vi "HFRR ADV v044.vi"() -> ()   [LabVIEW 2025] (continued)
  # "Calibration failed. The measured stroke length differs from the factory calibration value by more than 20%. Please perform the calibration again."
  # "Step 1 — Ball Holder"
  # "Remove the ball holder by loosening and removing the center screw for Friction calibration."
  # "Step 2 — Disc Holder"
  # "Remove the disc holder by loosening and removing the opposing screws. Clean any fluid present in the disc holder."
  # "Step 3 — Calibration Head"
  # "Place the calibration holder in position and securely tighten the center screw."
  # "Step 4 — Calibration Holder"
  # "Place the calibration holder in position and tighten the two securing screws"
  # "Step 5 — Tare (Spring at Free Length)"
  # "Ensure the spring is at its contact (compressed) length — the micrometer head is in contact. Click Tare Sensor to zero the friction force baseline."
  # "Step 6 — Measure Friction Force"
  # "Run the Actual Test to measure Friction Force."
  # "Calibration in Progress"
  # "Step 7 — CALIBRATION RESULT"
  # "Calibration completed successfully. The measured friction force is within the acceptable tolerance range of the factory calibration value."
  # "Calibration failed. The measured friction force differs from the factory calibration value . Please perform the calibration again."
  # "Spring Constant: k = 1.000 N/mm\nSpring force |F| = k Ч d"
  # "Calibrates the sample/bath temperature sensor. \nUsed for test specimen and lubricant temperature measurement."
  # "Calibrates the ambient air temperature sensor. \nUsed for environmental chamber monitoring."
  # "Set B\n60 °C\nHigh-point calibration"
  # "Set A\n0 °C\nIce-point calibration"
  # "Set B\n60 °C\nHigh-point calibration"
  # "Set A\n0 °C\nIce-point calibration"
  # "Select Temperature Sensor"
  # "Choose which temperature sensor you are calibrating. Both use the same two-\npoint procedure: 0 °C (ice-point) and 60 °C (high-point)."
  # "Step 1 — Reference Instrument Setup"
  # "Connect a calibrated reference to the DUT port. This calibration performs two sets: one at 0 °C and one at 60 °C."
  # "Set A\n0 °C\nIce-point calibration"
  # "Set B\n60 °C\nHigh-point calibration"
  # "Allow the temperature bath to stabilise for at least 2 minutes at each set-point before recording the reading."
  # "Step 2 — Set A:  0 °C Calibration"
  # "Connect the  0 °C reference connector. Wait for the temperature to stabilise. Once stable, and click Record Point."
  # "Step 3 — Set B:  60 °C Calibration"
  # "Connect the  60 °C reference connector. Wait for the temperature to stabilise. Once stable, and click Record Point."
  # "Sample Temperature Calibration Complete"
  # "Sample Temperature Calibration PASSED\nMax deviation 0.200 °C — within ±0.5 °C tolerance. Two-point correction applied (0 °C & 60 °C)."
  # "Sample  Temperature Calibration Failed\nmeasured Sample Temperature differs from the factory calibration value"
  # "Step 1 — Reference Instrument Setup"
  # "Connect a calibrated reference to the DUT port. This calibration performs two sets: one at 0 °C and one at 60 °C."
  # "Set A\n0 °C\nIce-point calibration"
  # "Set B\n60 °C\nHigh-point calibration"
  # "Allow the temperature bath to stabilise for at least 2 minutes at each set-point before recording the reading."
  # "Step 2 — Set A:  0 °C Calibration"
  # "Connect the  0 °C reference connector. Wait for the temperature to stabilise. Once stable, and click Record Point."
  # "Step 3 — Set B:  60 °C Calibration"
  # "Connect the  60 °C reference connector. Wait for the temperature to stabilise. Once stable, and click Record Point."
  # "Air Temperature Calibration Complete"
  # "Air Temperature Calibration PASSED\nMax deviation 0.200 °C — within ±0.5 °C tolerance. Two-point correction applied (0 °C & 60 °C)."
  # "Air  Temperature Calibration Failed\nmeasured Sample Temperature differs from the factory calibration value"
  # "System Control Commands\nS;1 - Starts the full automation cycle (Runs Priming-humidify till 70RH sequence first, then switches to Maintenance).\nS;0 - Stops the system immediately and enters Standby mode (Safe State: All actuators OFF).\nM;1 - Skips the priming sequence and jumps directly to Maintenance mode (PID control).\nR;1 - Resets the logic state machine and clears all errors, returning to Standby.\nService Mode (Manual Control)\nX;1 - Enters Manual Service Mode. This disables all automatic logic, sensor safety checks, and timers.\nX;0 - Exits Manual Service Mode and returns to Standby (Safe State).\nActuator Commands (Only work after sending X;1)\nP;[0-255] - Sets the Pump PWM. Note that this is Active Low (0 = Max Flow, 255 = Pump OFF).\nF;I;[0-255] - Sets the Intake Fan speed (0 = OFF, 255 = Max Speed).\nF;O;[0-255] - Sets the Exhaust Fan speed (0 = OFF, 255 = Max Speed).\nD;1 - Turns the Dehumidifier Relay ON.\nD;0 - Turns the Dehumidifier Relay OFF."
  # "%RH"
types:
  T1 = enum32{"Home", "Dashboard", "Imaging", "Report", "Analysis", "About", "Test Setup", "Advance", "Calibration"}
  T2 = typedef "imagedata.ctl" = cluster{"image type":i32, "image depth":i32, "image":u8[], "mask":u8[], "colors":u32[], "Rectangle":cluster{"left":i16, "top":i16, "right":i16, "bottom":i16}}
  T3 = enum32{"HOME", "Test Setup", "Acquire", "Compare Files", "Print Report", "About", "Advance", "Mooha"}
  T4 = enum32{"HOME", "Test Setup", "Acquire", "Adv Scar", "Adv Scar Report", "Compare Files", "Calibration", "About", "Advance", "Mooha"}
  T5 = enum16{"ASTM D6079", "ISO 12156", "CEC F-096-A-06", "Custom"}
  T6 = enum32{"Dashboard 1", "Dashboard 2", "Dashboard 3"}
  T7 = enum32{"COF", "Friction", "ECR", "Temperature", "Stroke"}
  T8 = enum32{"Coefficient Of Friction", "Air Temperature", "Humidity", "Stroke", "Sample Temperature", "Electrical Contact Resistance", "Frequency", "Air Temp vs Rh"}
  T9 = enum32{"Main", "Stroke", "Friction", "Temperature"}
  T10 = enum32{"Stroke Calibration", "Friction Force Calibration", "Temperature Calibration", "Default"}
  T11 = enum32{"Step 1", "Step 2", "Step 3", "Step 4", "Step 5", "Step 6", "Step 7", "Step 8", "Step 9"}
  T12 = enum32{"Test Progress", "Stroke Points Completed"}
  T13 = enum32{"Page 1", "Page 2", "Page 3", "Page 4", "Page 5", "Page 6"}
  T14 = enum32{"Main", "Step 1", "Step 2", "Step 3", "Step 4", "Air Step 1", "Air Step 2", "Air Step 3", "Air Step 4"}
  T15 = enum32{"Air Temperature", "Sample Temperature", "Default"}
  T16 = enum32{"COMMUNICATION", "CALIBRATION", "Temp Variables", "Camera", "WO 2472 (1)", "WO 2472 (2)", "WO 2472 (3)"}
  T17 = typedef "Auto Start enum.ctl" = enum16{"Init", "Humidity & Temperature On", "Reach point", "Maintain Stage", "Start Stage", "close", "Exit"}
  T18 = cluster{"Read Heave and Surge":string, "Bytes at Heave Port":dbl, "Heave and Surge COM Port:":refnum<visa-resource-name>, "Com Port 2":refnum<visa-resource-name>, "Residual Due":string, "Heave COM Status 2":bool, "Heave COM Status":bool, "Port 2":bool, "Sway PPR":dbl, "Surge PPR":dbl, "Heave PPR":dbl, "Sway Pitch":dbl, "Surge Pitch":dbl, "Heave Pitch":dbl, "Sway Pulses/mm":dbl, "Surge Pulses/mm":dbl, "Heave Pulses/mm":dbl, "inner loop":dbl, "Read Heave and Surge 2":string, "String 36":string, "Write S":bool, "WriteCC1":string[], "Heave COM Loop":i32, "LastCom":string, "EXIT":bool, "Error Heave":errorcluster}
  T19 = enum8{"Enabled", "Disabled", "Disabled and Grayed Out"}
  T20 = cluster{"Read Uno":string, "Bytes at Heave Port":dbl, "UNO COM Port:":refnum<visa-resource-name>, "UNO COM Port: 2":refnum<visa-resource-name>, "Residual Due":string, "UNO COM Status 2":bool, "UNO COM Status":bool, "Port 2":bool, "Sway PPR":dbl, "Surge PPR":dbl, "Heave PPR":dbl, "Sway Pitch":dbl, "Surge Pitch":dbl, "Heave Pitch":dbl, "Sway Pulses/mm":dbl, "Surge Pulses/mm":dbl, "Heave Pulses/mm":dbl, "inner loop":dbl, "Read Heave and Surge 2":string, "String 36":string, "Write S":bool, "WriteCC1":string[], "Heave COM Loop":i32, "LastCom":string, "EXIT":bool, "Error Heave":errorcluster}
  T21 = enum32{"HOME", "Test Setup", "Acquire", "Adv Scar", "Adv Scar Report", "Compare Files", "About", "Advance", "Mooha"}
  T22 = typedef "POST ANALYSIS ENUM.ctl" = enum16{"OPEN EXE", "INIT", "OPEN FILE", "FIT", "DRAW REC", "DRAW LINE", "PAN", "ZOOM IN", "ZOOM OUT", "SET ZOOM", "CLEAR ROI", "GET MEASUREMENTS", "RESIZE MODE", "STREAM START", "STREAM STOP", "SHOW UI", "MINIMIZE UI", "HIDE UI", "CKISE APP", "CLOSE CONNECTION", "SAVE IMAGE", "SET ROI COLOR", "READ", "TCP CHECK", "CLOSE"}
  T23 = typedef "CAMERA LIVE FEED ENUM.ctl" = enum16{"OPEN EXE", "INIT", "READ", "CAMERA CONNECT", "CAMERA START", "CAMERA STOP", "CAMERA GRAY", "CAMERA RGB", "CAMERA MINIMIZE", "CAMERA CLOSE", "CAMERA MODE LIST", "CAMERA MODE SET", "CAMERA RESTORE", "CAMERA SAVE", "CLOSE"}
  T24 = enum16{"Always On", "Always Off", "Off While Running"}
  T25 = enum32{"Home", "Dashboard", "Imaging", "Report", "Analysis", "About", "Test Setup", "Advance"}
  T26 = cluster{"File Name":string, "Test Method":string, "Operator":string, "Fuel Description":string, "Date and time":string}
  T27 = enum32{"Home", "Dashboard", "Imaging", "Report", "Analysis", "About", "Test Setup"}
  T28 = enum32{"HOME", "Test Setup", "Acquire", "Compare Files", "About", "Advance", "Mooha"}
  T29 = typedef "NI_ReportGenerationCore.lvlib/HTML Report Image Alignment.ctl" = enum16{"(default)", "LEFT", "RIGHT", "TOP", "TEXTTOP", "MIDDLE", "ABSMIDDLE", "BASELINE", "BOTTOM", "ABSBOTTOM"}
  T30 = cluster{"y":dbl, "LVDT STROKE DISPLAY":dbl, "y":dbl}
  T31 = enum16{"INIT", "READ", "MANUAL WRITE", "WRITE", "CLOSE", "ERROR INIT"}
diagram:
  w1 = FALSE
  w8 = 0.0 ("ch0_filt")
  w10 = -9999999.0 ("max_ch0")
  w11 = 9999999.0 ("min_ch0")
  w22 = FALSE ("Visible")
  w23 = T19."Enabled" ("Disabled")
  w26 = FALSE ("Visible")
  w25 = FALSE ("Humidity Off Command")
  w41 = "" ("USER ID")
  (unwired) T21."HOME" ("Main Tab")
  # "Temperature Continue Air Step 2"
  # "[CH1]    - FF\n[CH2]   - TEMPERATURE\n[CH3]    - Humidity\n[CH4]    - AIR TEMP\n[CH5]\\- Visa Uno\n[CH6] \\- Visa Due\n[CH7]  \\- file path\n[CH8]   - Displacement Gain\n[CHA]   - Stroke Gain\n[CHB]   - Stroke PID Gain\n[CHC]   -Language Selection\n[CHD]   -Power +\n[CHE]   -Power_\n[CHF]   -Heater\n[CHG]   -Humidity Wet\n[CHH]   -Humidity Dry\n[CHI]   -Integral Time \n[CHIJ   -Air intercept\n[CHI]   -Temp Intercept"
  n1 = local write "Cal Password"("" ("Cal Password")) -> ()
  n2 = property on="Auto Start Test" class="Bool (strict)"("Visible"=TRUE) -> ()  [unwired: 2 in, 2 out]
  n3 = property on="Friction Force Calibration Result Tab" class="TabCtl (strict)"("Visible"=FALSE) -> ()  [unwired: 2 in, 2 out]
  n4 = property on="FRICVALZ 2" class="Bool (strict)"("DisabledEnum"=w23) -> ()  [unwired: 2 in, 2 out]
  n5 = property on="FRICVALZ 4" class="Bool (strict)"("DisabledEnum"=w23) -> ()  [unwired: 2 in, 2 out]
  n6 = property on="FRICVALZ 3" class="Bool (strict)"("DisabledEnum"=w23) -> ()  [unwired: 2 in, 2 out]
  n7 = property on="About" class="Clust (strict)"("Visible"=FALSE) -> ()  [unwired: 2 in, 2 out]
  n8 = property on="Wrong Password" class="Str"("Visible"=w22) -> ()  [unwired: 2 in, 2 out]
  n9 = property on="Calibration 2" class="TabCtl (strict)"("Visible"=w22) -> ()  [unwired: 2 in, 2 out]
  n10 = local write "Temperature Selection"(T15."Default" ("Temperature Selection")) -> ()
  n11 = flat-sequence {
    tunnel: [w70] -> w7
    tunnel: [w115] -> w33
    tunnel: w7 -> [w110]
    tunnel: [w116] -> w35
    tunnel: w33 -> [w116]
    tunnel: w35 -> [w176]
    tunnel: [w176] -> w34
    tunnel: w34 -> [w207]
    tunnel: [w207] -> w44
    tunnel: w44 -> [w214]
    tunnel: [w220] -> w32
    tunnel: [w208] -> w31
    tunnel: [w262] -> w6
    tunnel: [w261] -> _
    tunnel: w32 -> [w261]
    tunnel: w31 -> [w262]
    frame #0 {
      n12 = call "CLOSE CONNECTION.vi"("error in (no error)"="error in (no error) 2") -> ("error out"=w75:errorcluster)  [unwired: 10 in]
      n13 = call <vilib>:"Clear Errors.vi"("error in (no error)"=w75) -> ("error out"=w74:errorcluster)  [unwired: 5 in, 1 out]
      n14 = disable-structure shown="Enabled" {
        disable-tunnel: w74 -> [w102 _]
        disable-tunnel: [w101 _] -> w73
        frame Enabled {
          n15 = call <userlib>:"Fit VI window to Largest Dec.vi"("error in (no error)"=w102, "border spacing (2 px)"=1) -> ("error out"=w105:errorcluster, "dup VI Ref"=w109:refnum<vi>)  [unwired: 4 in]
          n16 = invoke on="Invoke Node" class="VI" method="FP.Run-Time Position.Maximized"(reference=w109, error in=w105) -> (error out=w106:errorcluster)  [unwired: 2 in, 3 out]
          n17 = call <vilib>:"Clear Errors.vi"("error in (no error)"=w106) -> ("error out"=w108:errorcluster)  [unwired: 5 in, 1 out]
          n18 = control-ref of="This VI"() -> (w100:refnum<vi>)
          n19 = invoke on="Invoke Node" class="VI" method="Default Vals.Reinit All"(reference=w100, error in=w108) -> (reference out=w104:refnum<vi>, error out=w103:errorcluster)  [unwired: 1 in, 1 out]
          n20 = Close Reference(reference=w104, error in (no error)=w103) -> (error out=w101:errorcluster)
        }
        frame Disabled {
        }
      }
      n21 = call "Stall Data Flow.vim"("value in"=w73, "milliseconds to wait"=u32 2000) -> ("value out"=w72:errorcluster)  [unwired: 1 out]
      n22 = call "Read Config.vi"("error in (no error)"=w72) -> ("error out"=w70:errorcluster, "STROKE PARAMETERS"=w81:dbl[], "ADC PARAMETERS"=w82:dbl[], "PID  PARAMETERS"=w83:dbl[], "CALIBRATION PARAMETERS"=w68:string[], "Stroke Calibration"=w80:string)  [unwired: 5 in]
      n23 = Index Array(array=w81) -> (element #1=w98:dbl, element #2=w99:dbl)  [unwired: 2 in]
      n24 = Index Array(array=w68) -> (element #1=w67:string, element #2=w66:string, element #3=w65:string, element #4=w64:string, element #5=w63:string)  [unwired: 5 in]
      n25 = Index Array(array=w82) -> (element #1=w94:dbl, element #2=w95:dbl, element #3=w96:dbl, element #4=w97:dbl, element #5=w62:dbl)  [unwired: 5 in]
      n26 = Index Array(array=w83) -> (element #1=w85:dbl, element #2=w86:dbl, element #3=w87:dbl, element #4=w88:dbl, element #5=w89:dbl, element #6=w90:dbl, element #7=w91:dbl, element #8=w92:dbl, element #9=w93:dbl)  [unwired: 9 in]
      n27 = local write "STROKE FILTER"(w98) -> ()
      n28 = local write "Add up Stroke"(w99) -> ()
      n29 = local write "milliseconds to wait"(w85) -> ()
      n30 = local write "dt"(w86) -> ()
      n31 = local write "kp"(w87) -> ()
      n32 = local write "ki"(w88) -> ()
      n33 = local write "kd"(w89) -> ()
      n34 = local write "max_step_change"(w90) -> ()
      n35 = local write "max_amplitude"(w91) -> ()
      n36 = local write "min_amplitude"(w92) -> ()
      n37 = local write "startup_cmd"(w93) -> ()
      n38 = local write "VREF"(w94) -> ()
      n39 = local write "ADC_Resolution"(w95) -> ()
      n40 = local write "PIEZO_CAL_FACTOR"(w96) -> ()
      n41 = local write "NORMAL_FORCE"(w97) -> ()
      n42 = local write "Machine Serial Number"(w63) -> ()
      n43 = local write "STROKE CALIBRATION"(w67) -> ()
      n44 = local write "FRICTION CALIBRATION"(w66) -> ()
      n45 = local write "TEMPERATURE CALIBRATION"(w65) -> ()
      n46 = Fract/Exp String To Number(string=w64) -> (number=w69:dbl)  [unwired: 3 in, 1 out]
      n47 = local write "FF CAL EXCPTED VALUE"(w62) -> ()
      n48 = Spreadsheet String To Array(delimiter (Tab)=";", format string="", spreadsheet string=w80, array type (2D Dbl)=dbl[] []) -> (array=w84:dbl[])
      n49 = local write "Temperature diff"(w69) -> ()
      n50 = local write "calibration values"(w84) -> ()
    }
    frame #1 {
      n51 = property on="Auto Scar Check" class="Clust (strict)"("Visible"=TRUE) -> ()  [unwired: 2 in, 2 out]
      n52 = property on="Sign In" class="Bool (strict)"("DisabledEnum"=T19."Disabled" ("Disabled")) -> ()  [unwired: 2 in, 2 out]
      n53 = local write "sign in temp"(FALSE ("sign in temp")) -> ()
      n54 = call "dialog box.vi"("Status"="Before starting the test, verify that the microscope cable is connected.", "error in"=w110) -> ("error out"=w115:errorcluster)  [unwired: 8 in]
    }
    frame #2 {
      (unwired) TRUE ("Re-Initialise")
      # "kkkkk"
      # "C:\\Windows\\wndcm_pw_stdED hfrr.txt"
      # "C:\\LAB-IQ NXT"
      # "C:\\LAB-IQ NXT\\wndcm_pw_stdED hfrr.txt"
      # "password file"
      n55 = Current VI's Path() -> (path=w132:path)
      n56 = Strip Path(path=w132) -> (stripped path=w125:path)  [unwired: 1 out]
      n57 = local write "main tab sub"(enum32{"Page 1", "Page 2"}."Page 1" ("main tab sub")) -> ()
      n58 = local write "Main Tab Display"(T6."Dashboard 1" ("Main Tab Display")) -> ()
      n59 = local write "Main Tab"(T4."HOME" ("Main Tab")) -> ()
      n60 = Path To String(path=w125) -> (string=w127:string)
      n61 = Search/Split String(string=w127, search string/char (-)=".exe") -> (match + rest of string=w129:string)  [unwired: 1 in, 2 out]
      n62 = Match True/False String(2:".vi" ("false string"), 3:".exe" ("true string"), 4:w129) -> (0:w126:bool)  [unwired: 1 out]
      n63 = List Folder(path=path "C:/LAB-IQ" ("directory path"), pattern="*.txt") -> (filenames=w138:string[])  [unwired: 2 in, 3 out]
      n64 = case shown="True" w126 {
        tunnel: w125 -> [w147 w149]
        tunnel: [w147 w148] -> w123
        frame False {
        }
        frame True {
          n65 = Strip Path(path=w149) -> (stripped path=w148:path)  [unwired: 1 out]
        }
      }
      n66 = Search 1D Array(1D array=w138, element="wndcm_pw_stdED hfrr.txt") -> (index of element=w141:i32)  [unwired: 1 in]
      n67 = Equal?(x=w141, y=-1) -> (x = y?=w136:bool)
      n68 = Path To String(path=w123) -> (string=→"Gain path":string)
      n69 = case shown="True" w136 {
        frame False {
        }
        frame True {
          n70 = String To Byte Array(string="123\n") -> (unsigned byte array=w154:u8[])
          n71 = Array Size(array=w154) -> (size(s)=w153:i32)
          n72 = for {
            N: w153 -> [_]
            tunnel: w154 -> [w167]
            tunnel: [w164] -> w156 mode=indexing
            tunnel: w153 -> [w159]
            i -> [w157]
            n73 = Decrement(x=w159) -> (x-1=w160:i32)
            n74 = Index Array(array=w167, index=w157) -> (element=w166:u8)
            n75 = Equal?(x=w157, y=w160) -> (x = y?=w161:bool)
            n76 = Number To Decimal String(number=w166) -> (decimal integer string=w165:string)  [unwired: 1 in]
            n77 = Select(t="", s=w161, f="\r") -> (s? t:f=w158:string)
            n78 = Concatenate Strings(w165, w158) -> (w164:string)
          }
          n79 = local read "file path"() -> (w150:path)
          n80 = Concatenate Strings(w156) -> (w152:string)
          n81 = call <vilib>:"Write Characters To File.vi"("append to file? (new file:F)"=FALSE, "character string"=w152, "file path (dialog if empty)"=w150) -> ()  [unwired: 2 in, 1 out]
        }
      }
      n82 = local write "conststatus"(0.0 ("rpm value : 2")) -> ()
      n83 = local write "EVENT LOG"("") -> ()
      n84 = local write "COUNT"(0 ("COUNT")) -> ()
      n85 = local write "clk"(0.0 ("clk")) -> ()
      n86 = local write "Flag"(0.0 ("Flag")) -> ()
      n87 = local write "Lan flag"(0.0 ("Lan flag")) -> ()
      n88 = local write "Com flag"(u32 0 ("Com flag")) -> ()
      n89 = local write "refresh flag"(FALSE ("refresh flag")) -> ()
      "file path" <- path "C:/LAB-IQ/wndcm_pw_stdED hfrr.txt" ("file path")
      "FF buffer" <- dbl[] [] ("FF buffer")
    }
    frame #3 {
      # "C:\\WinDucom\\calibrate WO 2391.dcf"
      n90 = String To Path(string="C:\\LAB-IQ\\Image Calibrate v01.dcf") -> (path=w171:path)
      n91 = String To Path(string="C:\\LAB-IQ\\calibrate WO 2472.dcf") -> (path=w175:path)
      n92 = Open/Create/Replace File "Open File"(file path (use dialog)=w175) -> (refnum out=w174:refnum<file>)  [unwired: 5 in, 2 out]
      n93 = Open/Create/Replace File ("Open File")(file path (use dialog)=w171) -> (refnum out=w170:refnum<file>)  [unwired: 5 in, 2 out]
      n94 = for {
        N: 4 -> [_]
        tunnel: w170 -> [w182]
        i -> [w178]
        n95 = Read from Text File ("Read File")(file (use dialog)=w182) -> (text=w183:string)  [unwired: 3 in, 3 out]
        n96 = String Subset(string=w183, offset (0)=6, length (rest)=10 ("length (rest)")) -> (substring=w179:string)
        n97 = Fract/Exp String To Number(string=w179) -> (number=w177:dbl)  [unwired: 3 in, 1 out]
        n98 = case shown="3" w178 {
          tunnel: w177 -> [w184 w185 _ w186 _]
          frame 0 {
            n99 = local write "5x Gain"(w184) -> ()
          }
          frame 1 {
            n100 = local write "10x Gain"(w185) -> ()
          }
          frame 2 {
          }
          frame 3 {
            n101 = local write "100x gain"(w186) -> ()
          }
          frame 4, Default {
          }
        }
      }
      n102 = for {
        N: 24 -> [_]
        tunnel: w174 -> [w195]
        i -> [w189]
        (unwired) TRUE ("line mode (F)")
        n103 = Read from Text File "Read File"(file (use dialog)=w195) -> (text=w194:string)  [unwired: 3 in, 3 out]
        n104 = Match Pattern(string=w194, regular expression="]") -> (after substring=w192:string)  [unwired: 1 in, 3 out]
        n105 = String Subset(string=w194, offset (0)=5, length (rest)=10 ("length (rest)")) -> (substring=w187:string)
        n106 = Fract/Exp String To Number(string=w187) -> (number=w188:dbl)  [unwired: 3 in, 1 out]
        n107 = Match Pattern(string=w192, regular expression="-") -> (before substring=w190:string)  [unwired: 1 in, 3 out]
        n108 = case shown="18" w189 {
          tunnel: w188 -> [_ _ _ _ _ _ _ _ _ _ w202 _ _ _ _ _ _ _ _ _ _ _ _ _ _]
          tunnel: w190 -> [_ _ _ _ w198 w199 w200 _ _ _ _ _ _ _ _ _ _ _ _ _ w203 _ w204 w205 _]
          frame 0 {
          }
          frame 1 {
          }
          frame 2 {
          }
          frame 3 {
          }
          frame 4 {
            n109 = local write "Com Port 1"(w198) -> ()
          }
          frame 5 {
            n110 = local write "Com Port 2"(w199) -> ()
            n111 = local write "visa due"(w199) -> ()
          }
          frame 6 {
            n112 = String To Path(string=w200) -> (path=w201:path)
            n113 = local write "File Path"(w201) -> ()
          }
          frame 7 {
          }
          frame 8 {
          }
          frame 9 {
          }
          frame 10 {
            n114 = local write "Language Selection"(w202) -> ()
          }
          frame 11 {
          }
          frame 12 {
          }
          frame 13 {
          }
          frame 14 {
          }
          frame 15 {
          }
          frame 16 {
          }
          frame 17 {
          }
          frame 18 {
          }
          frame 21 {
          }
          frame 22 {
            n115 = local write "Com Port 3"(w203) -> ()
          }
          frame 23 {
          }
          frame 19 {
            n116 = local write "C3 :"(w204) -> ()
          }
          frame 20 {
            n117 = local write "Camera Port :"(w205) -> ()
          }
          frame 24, Default {
          }
        }
      }
    }
    frame #4 {
      n118 = Wait (ms)(milliseconds to wait=u32 1000) -> ()  [unwired: 1 out]
    }
    frame #5 {
      w223 = u32 2000 ("milliseconds to wait")
      w250 = u32 2000 ("milliseconds to wait")
      n119 = call "CAMERA LIVE FEED FGV.vi"("Enum - Menu"=CAMERA_LIVE_FEED_ENUM."OPEN EXE", "error in (no error)"=w214) -> ("error out"=w256:errorcluster)  [unwired: 8 in, 1 out]
      n120 = call "IMAGE ANALYSIS.vi"("Enum"=POST_ANALYSIS_ENUM."OPEN EXE", "error in"=w214) -> ("error out"=w211:errorcluster)  [unwired: 8 in, 1 out]
      n121 = call "Stall Data Flow.vim"("value in"=w256, "milliseconds to wait"=w250) -> ("value out"=w254:errorcluster)  [unwired: 1 out]
      n122 = call "Stall Data Flow.vim"("value in"=w211, "milliseconds to wait"=u32 8000) -> ("value out"=w210:errorcluster)  [unwired: 1 out]
      n123 = call "CAMERA LIVE FEED FGV.vi"("Enum - Menu"=CAMERA_LIVE_FEED_ENUM."INIT", "error in (no error)"=w254) -> ("error out"=w252:errorcluster)  [unwired: 8 in, 1 out]
      n124 = call "IMAGE ANALYSIS.vi"("Enum"=POST_ANALYSIS_ENUM."INIT", "error in"=w210) -> ("error out"=w208:errorcluster)  [unwired: 8 in, 1 out]
      n125 = case shown="Error .." w252 {
        selector: w252 -> [w257 _]
        tunnel: [w257 _] -> w251
        frame No Error {
        }
        frame Error {
          n126 = One Button Dialog(message="Camera initialization error.\nPlease Restart the software") -> ()  [unwired: 1 in, 1 out]
        }
      }
      n127 = property on="Camera Port :" class="CmbBox"() -> ("Strings[]"=w248:string[], "Value"=w249:string)  [unwired: 2 in, 2 out]
      n128 = Search 1D Array(1D array=w248, element=w249) -> (index of element=w247:i32)  [unwired: 1 in]
      n129 = Type Cast(type=30, x=w247) -> (*(type *) &x=w245:i32)
      n130 = call "Stall Data Flow.vim"("value in"=w251, "milliseconds to wait"=w250) -> ("value out"=w227:errorcluster)  [unwired: 1 out]
      n131 = Add(x=w245, y=48) -> (x+y=w226:i32)
      n132 = call "CAMERA LIVE FEED FGV.vi"("Enum - Menu"=CAMERA_LIVE_FEED_ENUM."CAMERA CONNECT", "error in (no error)"=w227, "CAMERA PORT"=w226) -> ("error out"=w236:errorcluster)  [unwired: 7 in, 1 out]
      n133 = call "Stall Data Flow.vim"("value in"=w236, "milliseconds to wait"=u32 5000) -> ("value out"=w237:errorcluster)  [unwired: 1 out]
      n134 = call "CAMERA LIVE FEED FGV.vi"("Enum - Menu"=CAMERA_LIVE_FEED_ENUM."CAMERA MODE LIST", "error in (no error)"=w237) -> ("error out"=w239:errorcluster)  [unwired: 8 in, 1 out]
      n135 = call "Stall Data Flow.vim"("value in"=w239, "milliseconds to wait"=w223) -> ("value out"=w238:errorcluster)  [unwired: 1 out]
      n136 = call "CAMERA LIVE FEED FGV.vi"("Enum - Menu"=CAMERA_LIVE_FEED_ENUM."READ", "error in (no error)"=w238) -> ("error out"=w225:errorcluster, "data out"=→"Camera List":string)  [unwired: 8 in]
      n137 = Type Cast(type=30, x=0) -> (*(type *) &x=w219:i32)
      n138 = call "Stall Data Flow.vim"("value in"=w225, "milliseconds to wait"=w223) -> ("value out"=w224:errorcluster)  [unwired: 1 out]
      n139 = Add(x=w219, y=48) -> (x+y=w217:i32)
      n140 = call "CAMERA LIVE FEED FGV.vi"("Enum - Menu"=CAMERA_LIVE_FEED_ENUM."CAMERA MODE SET", "error in (no error)"=w224, "CAMERA MODE"=w217) -> ("error out"=w221:errorcluster)  [unwired: 7 in, 1 out]
      n141 = call "Stall Data Flow.vim"("value in"=w221, "milliseconds to wait"=u32 2000) -> ("value out"=w241:errorcluster)  [unwired: 1 out]
      n142 = call "CAMERA LIVE FEED FGV.vi"("Enum - Menu"=CAMERA_LIVE_FEED_ENUM."CAMERA START", "error in (no error)"=w241) -> ("error out"=w242:errorcluster)  [unwired: 8 in, 1 out]
      n143 = call "Stall Data Flow.vim"("value in"=w242, "milliseconds to wait"=u32 1000) -> ("value out"=w243:errorcluster)  [unwired: 1 out]
      n144 = call "CAMERA LIVE FEED FGV.vi"("Enum - Menu"=CAMERA_LIVE_FEED_ENUM."CAMERA MINIMIZE", "error in (no error)"=w243) -> ("error out"=w220:errorcluster)  [unwired: 8 in, 1 out]
    }
    frame #6 {
      n145 = case shown="No Error" w261 {
        frame No Error {
          n146 = property on="Auto Scar Check" class="Clust (strict)"("Visible"=FALSE) -> ()  [unwired: 2 in, 2 out]
        }
        frame Error {
        }
      }
      n147 = property on="Sign In" class="Bool (strict)"("DisabledEnum"=T19."Enabled" ("Disabled")) -> ()  [unwired: 2 in, 2 out]
      n148 = local write "sign in temp"(TRUE ("sign in temp")) -> ()
    }
  }
  n149 = local write "Calibration Selection"(T10."Default" ("Calibration Selection")) -> ()
  n150 = local write "SCAR MEASURMENT"(enum32{"Auto Scar", "Manual Scar"}."Manual Scar" ("SCAR MEASURMENT")) -> ()
  n151 = property on="Service Left" class="Bool (strict)"("Visible"=w1) -> ()  [unwired: 2 in, 2 out]
  n152 = property on="Service Right" class="Bool (strict)"("Visible"=w1) -> ()  [unwired: 2 in, 2 out]
  n153 = property on="Service Bottom" class="Bool (strict)"("Visible"=w1) -> ()  [unwired: 2 in, 2 out]
  n154 = local write "Temperature Off Command"(w25) -> ()
  n155 = local write "Main Dashboard Buttons"(T1."Home" ("Main Dashboard Buttons")) -> ()
  n156 = property on="Tab Control 6" class="TabCtl (strict)"("Visible"=FALSE) -> ()  [unwired: 2 in, 2 out]
  n157 = local write "Humidity Off Command"(w25) -> ()
  n158 = local write "CAMERA ROI MIN TEMP"(w25) -> ()
  n159 = local write "TEST FILE NAM,E SAVED"(w25) -> ()
  n160 = local write "LIVE FEED MIN TEMP"(w25) -> ()
  n161 = local write "SCAR MEASURMENT"(enum32{"Auto Scar", "Manual Scar"}."Manual Scar" ("SCAR MEASURMENT")) -> ()
  n162 = local write "Auto stop temp"(w26) -> ()
  n163 = local write "main tab sub"(enum32{"Page 1", "Page 2"}."Page 1" ("main tab sub")) -> ()
  n164 = while {
    stop <- w276 stop-if-true
    n165 = local read "Ambient Temperature"() -> (w274:dbl)
    n166 = local read "Sample Temperature 2"() -> (w273:dbl)
    n167 = Wait (ms)(milliseconds to wait=u32 200) -> ()  [unwired: 1 out]
    n168 = local write "Sensor value"(w274) -> ()
    n169 = local write "Sensor value"(w274) -> ()
    n170 = local write "Sensor value"(w273) -> ()
    n171 = local write "Sensor value"(w273) -> ()
    n172 = local write "Temperature — Live (Set A: 0 °C)"(w274) -> ()
    n173 = local write "Temperature — Live (Set A: 60 °C)"(w274) -> ()
    n174 = local write "Temperature — Live (Set A: 60 °C)"(w273) -> ()
    n175 = local write "Temperature — Live (Set A: 0 °C)"(w273) -> ()
    n176 = case shown="True" "Save Button" {
      selector: "Save Button" -> [_ w332]
      frame False {
      }
      frame True {
        n177 = Not(x=w332) -> (.not. x?=w331:bool)
        n178 = local read "Temperature diff"() -> (w328:dbl)
        n179 = local read "Machine Serial Number"() -> (w317:string)
        n180 = local read "milliseconds to wait"() -> (w364:u32)
        n181 = local write "Save Button"(w331) -> ()
        n182 = local read "max_step_change"() -> (w369:dbl)
        n183 = local read "FF CAL EXCPTED VALUE"() -> (w315:dbl)
        n184 = local read "max_amplitude"() -> (w370:dbl)
        n185 = local read "min_amplitude"() -> (w371:dbl)
        n186 = local read "PIEZO_CAL_FACTOR"() -> (w375:dbl)
        n187 = local read "startup_cmd"() -> (w372:dbl)
        n188 = local read "NORMAL_FORCE"() -> (w376:dbl)
        n189 = local read "ADC_Resolution"() -> (w374:dbl)
        n190 = local read "kp"() -> (w366:dbl)
        n191 = local read "kd"() -> (w368:dbl)
        n192 = local read "calibration values"() -> (w379:dbl[])
        n193 = local read "dt"() -> (w365:dbl)
        n194 = local read "ki"() -> (w367:dbl)
        n195 = local read "STROKE FILTER"() -> (w377:i32)
        n196 = local read "Add up Stroke"() -> (w378:dbl)
        n197 = Number To Fractional String(number=w328) -> (F-format string=w327:string)  [unwired: 3 in]
        n198 = local read "VREF"() -> (w373:dbl)
        n199 = Insert Into Array(array=dbl[] [], new element #1=w364, new element #2=w365, new element #3=w366, new element #4=w367, new element #5=w368, new element #6=w369, new element #7=w370, new element #8=w371, new element #9=w372) -> (w380:dbl[])  [unwired: 1 in]
        n200 = Insert Into Array(array=dbl[] [], new element #1=w373, new element #2=w374, new element #3=w375, new element #4=w376, new element #5=w315) -> (w381:dbl[])  [unwired: 1 in]
        n201 = Array To Spreadsheet String(delimiter (Tab)=";", array=w379, 3:"" ("format string")) -> (spreadsheet string=w383:string)
        n202 = Insert Into Array(array=dbl[] [], new element #1=w377, new element #2=w378) -> (w382:dbl[])  [unwired: 1 in]
        n203 = Insert Into Array(array=string[] [], new element #1="STROKE CALIBRATION", new element #2="FRICTION CALIBRATION", new element #3="TEMPERATURE CALIBRATION", new element #4=w327, new element #5=w317) -> (w329:string[])  [unwired: 1 in]
        n204 = call "Write Config.vi"("Stroke Calibration"=w383, "CALIBRATION PARAMETERS"=w329, "STROKE PARAMETERS"=w382, "ADC PARAMETERS"=w381, "PID  PARAMETERS"=w380) -> ("error out"=w362:errorcluster)  [unwired: 5 in, 1 out]
        n205 = call "Stall Data Flow.vim"("value in"=w362, "milliseconds to wait"=u32 2000) -> ("value out"=w363:errorcluster)  [unwired: 1 out]
        n206 = call "Read Config.vi"("error in (no error)"=w363) -> ("STROKE PARAMETERS"=w360:dbl[], "ADC PARAMETERS"=w359:dbl[], "PID  PARAMETERS"=w358:dbl[], "CALIBRATION PARAMETERS"=w323:string[], "Stroke Calibration"=w361:string)  [unwired: 5 in, 1 out]
        n207 = Index Array(array=w358) -> (element #1=w356:dbl, element #2=w355:dbl, element #3=w354:dbl, element #4=w353:dbl, element #5=w352:dbl, element #6=w351:dbl, element #7=w350:dbl, element #8=w349:dbl, element #9=w348:dbl)  [unwired: 9 in]
        n208 = Index Array(array=w359) -> (element #1=w347:dbl, element #2=w346:dbl, element #3=w345:dbl, element #4=w344:dbl, element #5=w314:dbl)  [unwired: 5 in]
        n209 = Index Array(array=w360) -> (element #1=w343:dbl, element #2=w342:dbl)  [unwired: 3 in, 1 out]
        n210 = Index Array(array=w323) -> (element #1=w320:string, element #2=w319:string, element #3=w318:string, element #4=w322:string, element #5=w316:string)  [unwired: 5 in]
        n211 = Spreadsheet String To Array(delimiter (Tab)=";", format string="", spreadsheet string=w361, array type (2D Dbl)=dbl[] []) -> (array=w357:dbl[])
        n212 = local write "STROKE CALIBRATION"(w320) -> ()
        n213 = local write "FRICTION CALIBRATION"(w319) -> ()
        n214 = local write "TEMPERATURE CALIBRATION"(w318) -> ()
        n215 = Fract/Exp String To Number(string=w322) -> (number=w321:dbl)  [unwired: 3 in, 1 out]
        n216 = local write "Machine Serial Number"(w316) -> ()
        n217 = local write "STROKE FILTER"(w343) -> ()
        n218 = local write "Add up Stroke"(w342) -> ()
        n219 = local write "VREF"(w347) -> ()
        n220 = local write "ADC_Resolution"(w346) -> ()
        n221 = local write "PIEZO_CAL_FACTOR"(w345) -> ()
        n222 = local write "NORMAL_FORCE"(w344) -> ()
        n223 = local write "FF CAL EXCPTED VALUE"(w314) -> ()
        n224 = local write "calibration values"(w357) -> ()
        n225 = local write "milliseconds to wait"(w356) -> ()
        n226 = local write "dt"(w355) -> ()
        n227 = local write "kp"(w354) -> ()
        n228 = local write "ki"(w353) -> ()
        n229 = local write "kd"(w352) -> ()
        n230 = local write "max_step_change"(w351) -> ()
        n231 = local write "max_amplitude"(w350) -> ()
        n232 = local write "min_amplitude"(w349) -> ()
        n233 = local write "startup_cmd"(w348) -> ()
        n234 = local write "Temperature diff"(w321) -> ()
      }
    }
    n235 = local read "USER ID"() -> (w271:string)
    n236 = local read "run test Calibration"() -> (w269:bool)
    n237 = disable-structure shown="Enabled" {
      disable-tunnel: [w283 w294] -> w270
      frame Disabled {
        n238 = local read "Point 1 - 0.2 mm"() -> (w293:bool)
        n239 = local read "Point 2 - 0.4 mm"() -> (w292:bool)
        n240 = local read "Point 3 - 0.6 mm"() -> (w291:bool)
        n241 = local read "Point 4 - 0.8 mm"() -> (w290:bool)
        n242 = local read "Point 5 - 1.0 mm"() -> (w289:bool)
        n243 = local read "Point 6 - 1.2 mm"() -> (w288:bool)
        n244 = And(x=w293, y=w292) -> (x .and. y?=w287:bool)
        n245 = And(x=w291, y=w290) -> (x .and. y?=w286:bool)
        n246 = And(x=w289, y=w288) -> (x .and. y?=w284:bool)
        n247 = And(x=w287, y=w286) -> (x .and. y?=w285:bool)
        n248 = And(x=w285, y=w284) -> (x .and. y?=w283:bool)
      }
      frame Enabled {
        n249 = local read "Point 5 - 1.0 mm"() -> (w294:bool)
      }
    }
    n250 = local read "START TEMP"() -> (w268:bool)
    n251 = local write "tested by 2"(w271) -> ()
    n252 = And(x=w268, y=w269) -> (x .and. y?=w267:bool)
    n253 = case shown="True" w267 {
      frame False {
        w295 = TRUE ("PAUSE")
        n254 = call "ELAPSED TIMER VI - Calibration.vi"("RESET"=w295, "PAUSE"=w295) -> ()  [unwired: 7 in, 3 out]
      }
      frame True {
        w298 = FALSE ("PAUSE")
        n255 = call "ELAPSED TIMER VI - Calibration.vi"("TARGET"=60.0, "RESET"=w298, "PAUSE"=w298) -> ("ELAPSED INDICATION"=w296:bool)  [unwired: 6 in, 2 out]
        n256 = case shown="False" w296 {
          frame False {
            n257 = local write "Friction Force Calibration Result Tab"(enum32{"Calibration Results", "Page 2"}."Calibration Results" ("Friction Force Calibration Result Tab")) -> ()
            n258 = property on="Friction Force Calibration Result Tab" class="TabCtl (strict)"("Visible"=FALSE) -> ()  [unwired: 2 in, 2 out]
          }
          frame True {
            n259 = stacked-sequence {
              frame #0 {
                n260 = local read "Friction"() -> (→"Friction cal":dbl)
                n261 = local write "run test Calibration"(FALSE ("run test Calibration")) -> ()
                n262 = local write "START TEMP"(FALSE ("START TEMP")) -> ()
              }
              frame #1 {
                n263 = Wait (ms)(milliseconds to wait=u32 1500) -> ()  [unwired: 1 out]
              }
              frame #2 {
                n264 = local write "Due Write"("VC;0") -> ()
              }
              frame #3 {
                n265 = Wait (ms)(milliseconds to wait=u32 1500) -> ()  [unwired: 1 out]
              }
              frame #4 {
                n266 = local write "Due Write"("VC;0") -> ()
              }
              frame #5 {
                n267 = property on="Friction Force Calibration Result Tab" class="TabCtl (strict)"("Visible"=TRUE) -> ()  [unwired: 2 in, 2 out]
                n268 = property on="Tab Control 6" class="TabCtl (strict)"("Visible"=FALSE) -> ()  [unwired: 2 in, 2 out]
              }
            }
          }
        }
      }
    }
    n269 = local read "Friction cal"() -> (w266:dbl)
    n270 = case shown="False" w270 {
      frame False {
        n271 = property on="Accept & Save" class="Bool (strict)"("DisabledEnum"=T19."Disabled" ("Disabled")) -> ()  [unwired: 2 in, 2 out]
        n272 = property on="Tab Control 5" class="TabCtl (strict)"("Value"=enum32{"OK", "NG"}."NG" ("Tab Control 5")) -> ()  [unwired: 2 in, 2 out]
      }
      frame True {
        n273 = property on="Accept & Save" class="Bool (strict)"("DisabledEnum"=T19."Enabled" ("Disabled")) -> ()  [unwired: 2 in, 2 out]
        n274 = property on="Tab Control 5" class="TabCtl (strict)"("Value"=enum32{"OK", "NG"}."OK" ("Tab Control 5")) -> ()  [unwired: 2 in, 2 out]
      }
    }
    n275 = Greater Or Equal?(x=w266, y="FF CAL EXCPTED VALUE") -> (x >= y?=w264:bool)
    n276 = case shown="False" w264 {
      selector: w264 -> [w277 w280]
      frame False {
        n277 = local write "FF PASS"(w277) -> ()
        n278 = local write "Friction Force result Tab"(enum32{"OK", "NG"}."NG" ("Friction Force result Tab")) -> ()
        n279 = property on="Accept & Save FF" class="Bool (strict)"("DisabledEnum"=T19."Disabled" ("Disabled")) -> ()  [unwired: 2 in, 2 out]
      }
      frame True {
        n280 = local write "Friction Force result Tab"(enum32{"OK", "NG"}."OK" ("Friction Force result Tab")) -> ()
        n281 = property on="Accept & Save FF" class="Bool (strict)"("DisabledEnum"=T19."Enabled" ("Disabled")) -> ()  [unwired: 2 in, 2 out]
        "FF PASS" <- w280
      }
    }
    n282 = local read "Quit"() -> (w276:bool)
  }
  n283 = local write "USERNAME"(w41) -> ()
  n284 = local write "Main Tab"(T4."HOME" ("Main Tab")) -> ()
  n285 = local write "USER ID"(w41) -> ()
  n286 = property on="Auto Scar Check  2" class="Clust (strict)"("Visible"=w26) -> (error out=w29:errorcluster)  [unwired: 2 in, 1 out]
  n287 = property on="Quit" class="Bool (strict)"("Value"=FALSE ("Quit")) -> (error out=w43:errorcluster)  [unwired: 2 in, 1 out]
  n288 = while {
    stop <- w384 stop-if-true
    n289 = event shown="[3] \"Auto\": Value Change" {
      selector: _ -> [_ _ _ _ _ _ _ _ _ _ _ _ _ _ _ _ _ _ _ _ _ _ _ _ _ _ _ _ _ _ _ _ _ _ _ _ _ _ _ _ _ _ _ _ _ _ _ _ _ _ _ _ _ _ _ _ _]
      dyn-events: _ -> [_ _ _ _ _ _ _ _ _ _ _ _ _ _ _ _ _ _ _ _ _ _ _ _ _ _ _ _ _ _ _ _ _ _ _ _ _ _ _ _ _ _ _ _ _ _ _ _ _ _ _ _ _ _ _ _ _]
      timeout: 100 -> [_ _ _ _ _ _ _ _ _ _ _ _ _ _ _ _ _ _ _ _ _ _ _ _ _ _ _ _ _ _ _ _ _ _ _ _ _ _ _ _ _ _ _ _ _ _ _ _ _ _ _ _ _ _ _ _ _]
      tunnel: [FALSE FALSE FALSE _ FALSE _ _ _ _ _ _ _ _ _ _ _ _ _ _ _ _ _ _ _ _ _ _ _ _ _ _ _ _ _ _ _ _ _ _ _ _ _ _ _ _ _ _ _ _ _ _ _ _ _ _ _ TRUE] -> w384
      event Timeout {
        n290 = event-data() -> ()  [unwired: 1 in, 3 out]
        n291 = disable-structure shown="Disabled" {
          frame Disabled {
            n292 = local read "Auto Start Test"() -> (w398:bool)
            n293 = local read "RUN"() -> (w399:bool)
            n294 = Or(x=w399, y=w398) -> (x .or. y?=w397:bool)
            n295 = case shown="True" w397 {
              frame False {
                w400 = TRUE ("PAUSE")
                n296 = call "ELAPSED TIMER VI - abort test.vi"("RESET"=w400, "PAUSE"=w400) -> ()  [unwired: 7 in, 3 out]
              }
              frame True {
                n297 = local read "Stroke 2"() -> (w405:dbl)
                n298 = local read "FF 3"() -> (w407:dbl)
                n299 = Equal?(x=w405, y=0.95 ("Stroke 2")) -> (x = y?=w402:bool)
                n300 = Equal?(x=w407, y=0.0 ("FF 3")) -> (x = y?=w403:bool)
                n301 = Or(x=w403, y=w402) -> (x .or. y?=w401:bool)
                n302 = case shown="True" w401 {